vi "Main - 副本.vi"() -> ()   [LabVIEW 2020]
uses:
  System.Windows.Forms
  Global_Variable/Global.vi
  Database/Global1.vi
  <userlib>/_MGI/Menu Building/MenuTypes/MenuStrip/MGI_MenuStrip.lvclass
  <userlib>/_MGI/Menu Building/MenuItemStatusChange/MGI_MenuItemStatusChange.lvclass
panel:
  out "上序状态":string
  in  "表格控件":string[][](table)
  in  "Andon":enum32{"未选择", "缺料报警", "质量报警", "故障报警"}(radio)
  in  "菜单":refnum<k24>(container)
  out "试验计时":u16
  out "工位传感器码":string
  out "生产数量":i32
  out "合格数量":i32
  out "userStatus":string caption="用户状态"
  out "userName":string caption="用户名"
  out "connectionMode":string caption="联机类型"
  out "产品型号":string
  in  "更换产品":refnum<vi>
  out "提示信息":string
  out "错误":bool
  out "时间字符串":string
  out "日期字符串":string
  out "自动":bool
  # "上转向轴组件压装"
  # "实验项目"
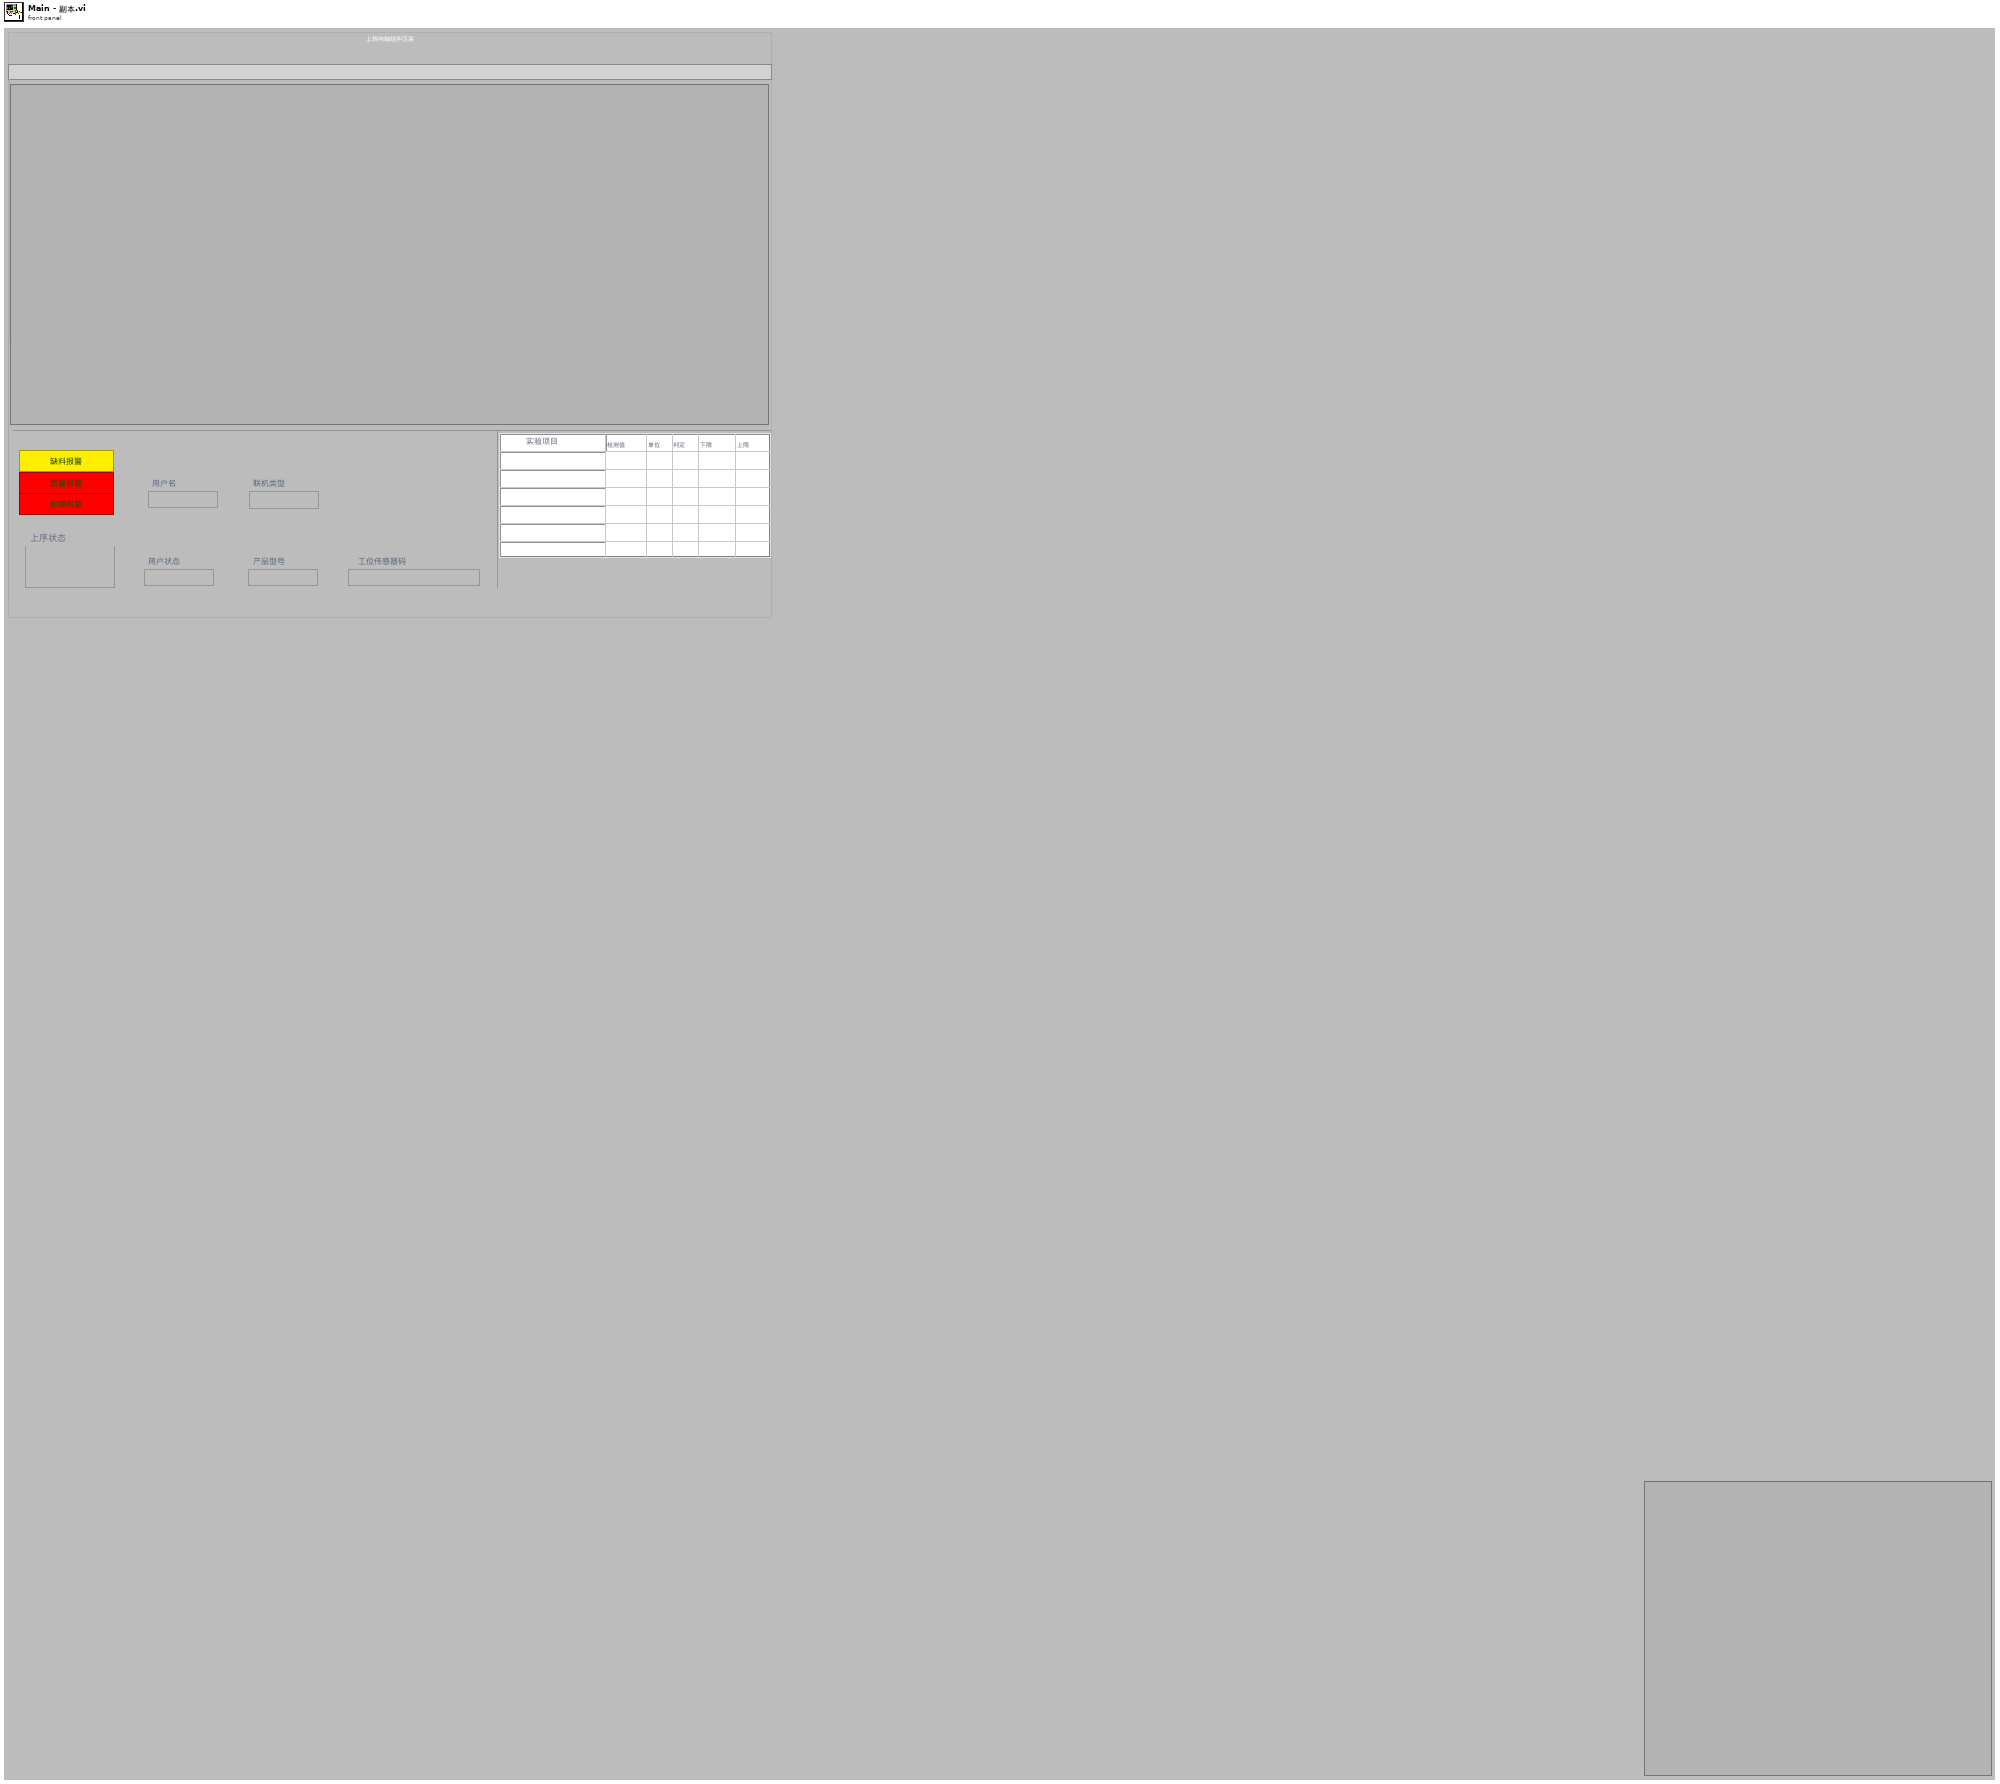
[diagram p1: front panel]
types:
  T1 = enum32{"Invalid", "Standard", "Closed", "Hidden", "Minimized", "Maximized"}
  T2 = cluster{"设备名称":string, "操作人员":string, "设备状态":enum16{"设备离线", "设备正常", "设备缺料", "设备故障", "质量报警"}, "附加信息":string}
  T3 = enum32{"invalid app kind", "Development System", "Run Time System", "Student Edition", "Embedded LabVIEW", "Evaluation", "Custom"}
  T4 = cluster{"用户编号":string, "用户名":string, "用户密码(密文)":string, "用户权限":string}
  T5 = cluster{"Core":cluster{"Current VI Reference":refnum<vi>, "Close Panel on Exit?":bool}, "Your Boolean data":bool, "Your string data":string}
  T6 = cluster{"Current VI Reference":refnum<vi>, "Close Panel on Exit?":bool}
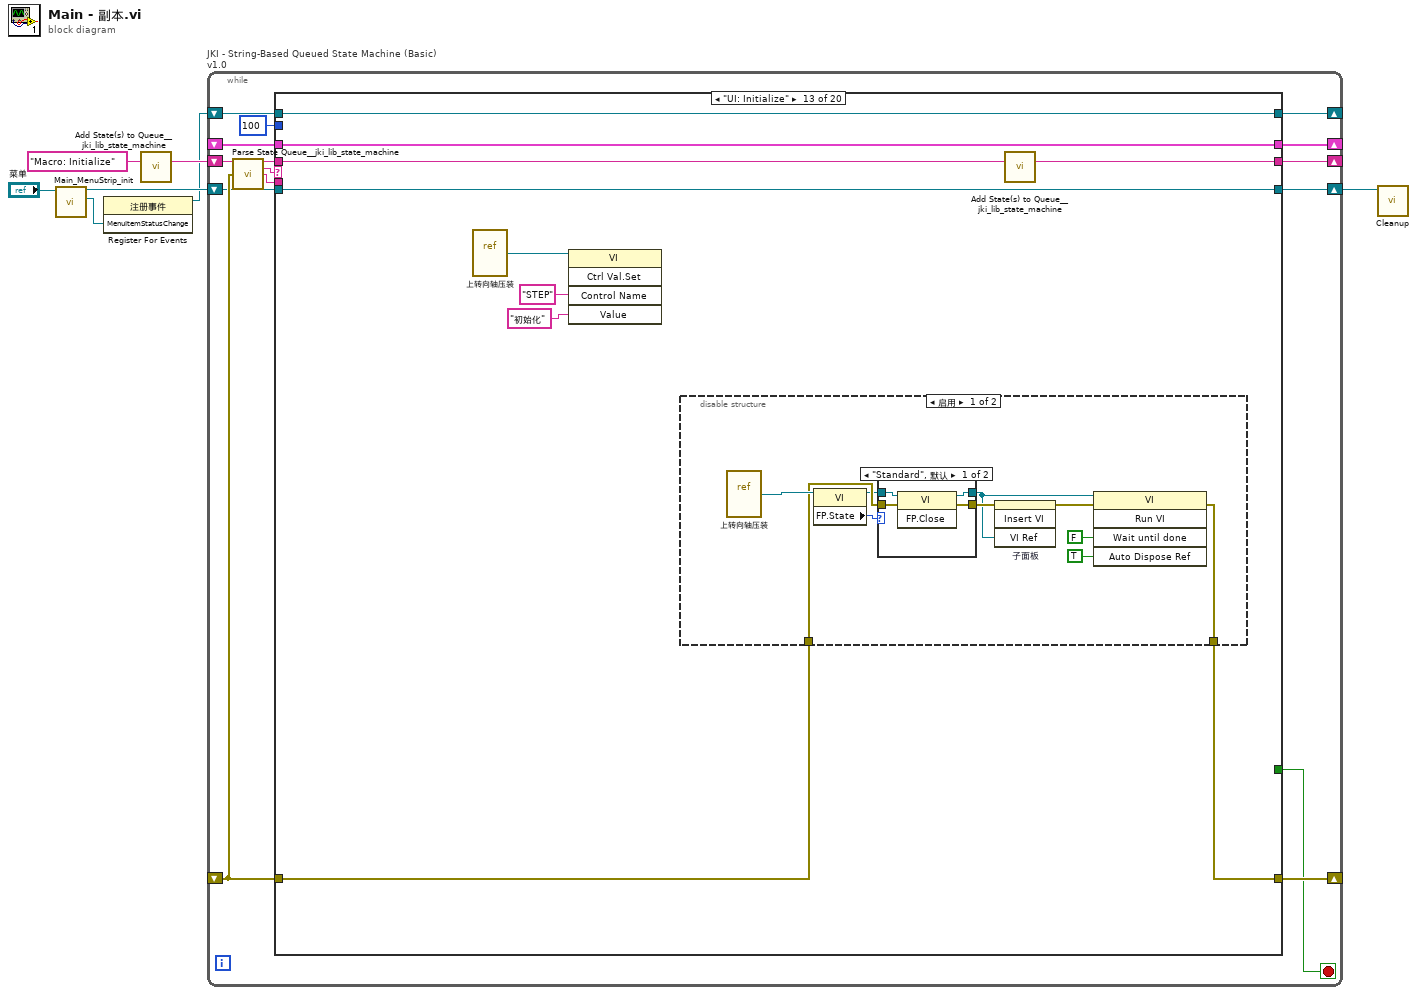
[diagram p0: block diagram]
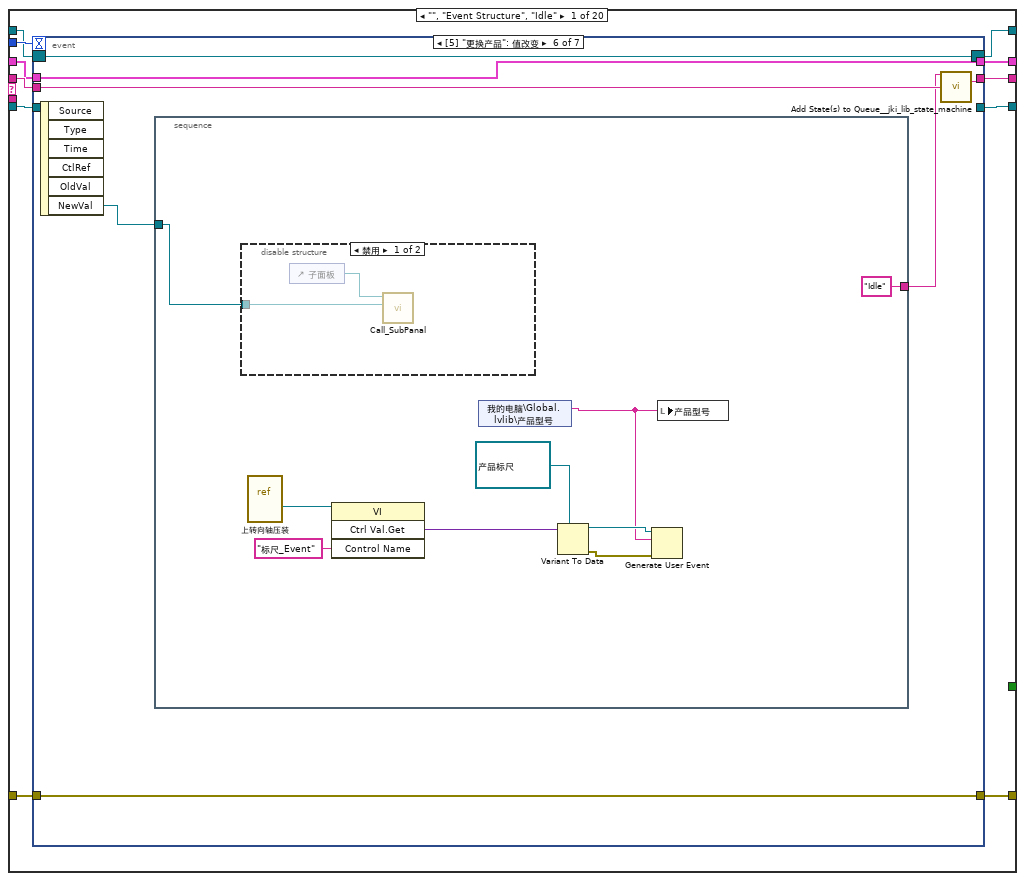
[diagram p2: hidden frame]
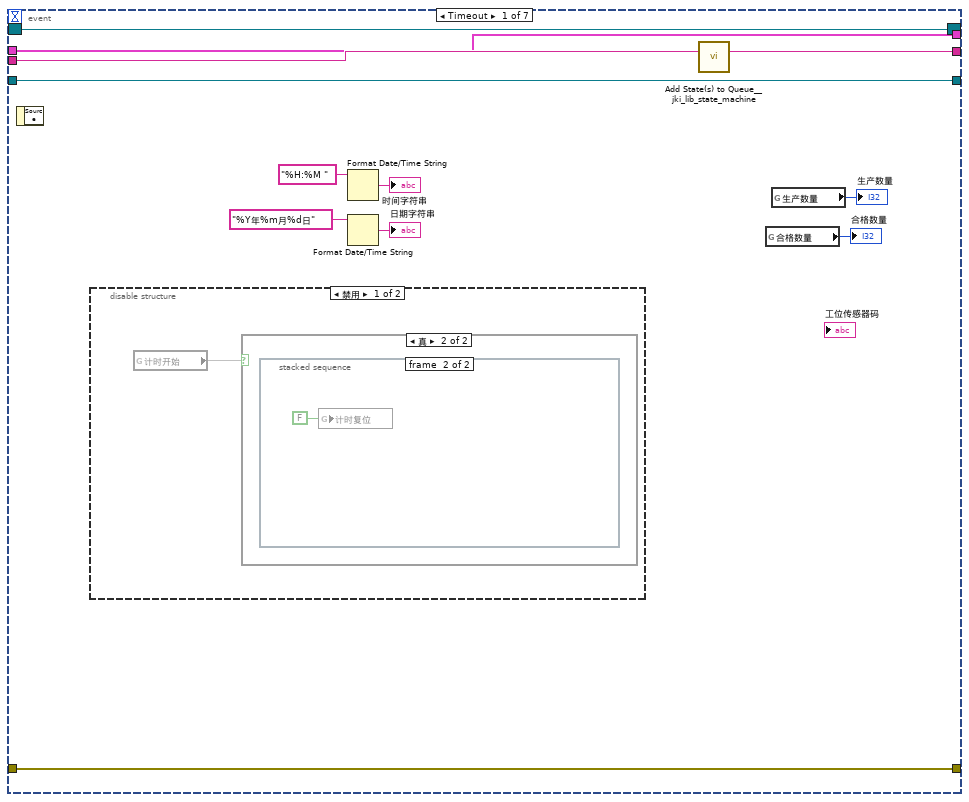
[diagram p3: hidden frame]
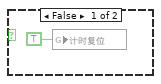
[diagram p4: hidden frame]
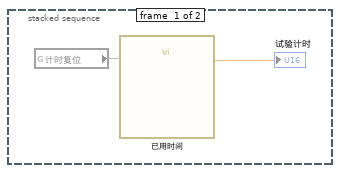
[diagram p5: hidden frame]
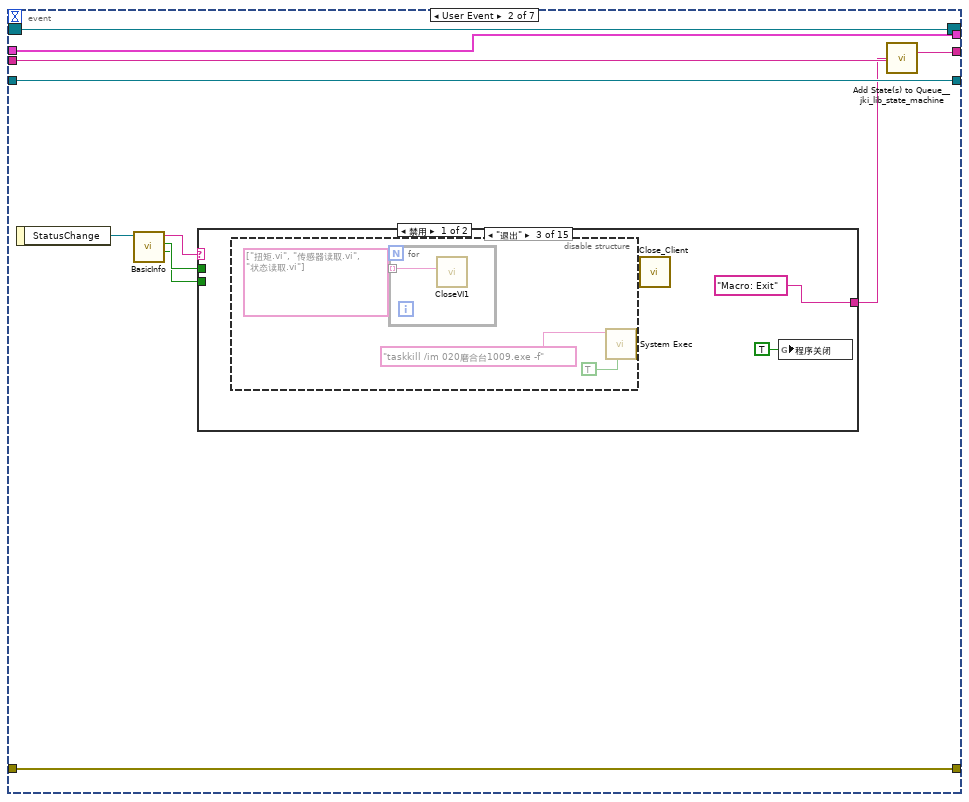
[diagram p7: hidden frame]
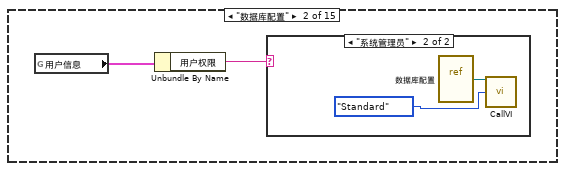
[diagram p9: hidden frame]
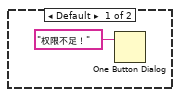
[diagram p10: hidden frame]
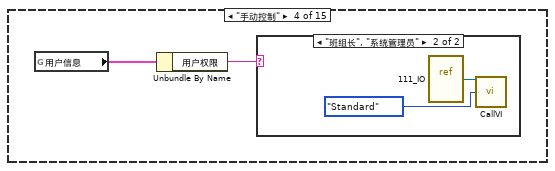
[diagram p12: hidden frame]
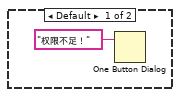
[diagram p13: hidden frame]
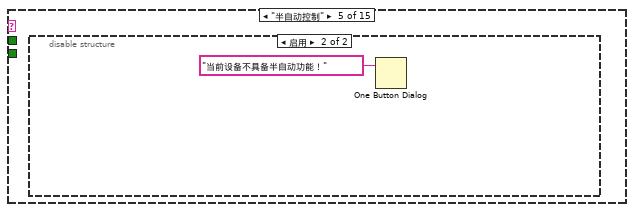
[diagram p14: hidden frame]
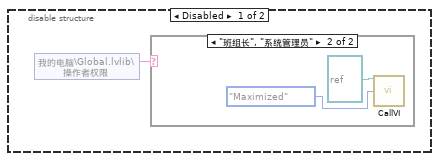
[diagram p15: hidden frame]
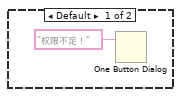
[diagram p16: hidden frame]
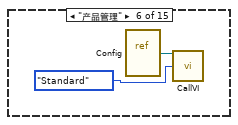
[diagram p17: hidden frame]
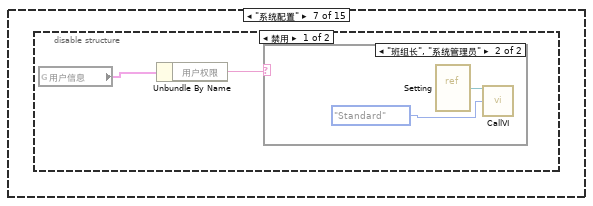
[diagram p18: hidden frame]
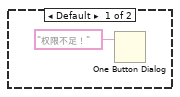
[diagram p19: hidden frame]
diagram:
  n1 = call "Main_MenuStrip_init.vi"("MenuStrip"="菜单") -> ("MenuItemStatusChange"=w2:refnum<user-event>, "Menu out"=w4:refnum<class "MGI_MenuStrip.lvclass">)  [unwired: 9 in]
  n2 = register-events(w2) -> (reference out=w1:refnum<event-registration>)  [unwired: 2 in, 1 out]
  n3 = call <vilib>:"Add State(s) to Queue__jki_lib_state_machine.vi"("State(s) in (\"\")"="Macro: Initialize") -> ("States Out"=w7:string)  [unwired: 14 in]
  n4 = while "JKI - String-Based Queued State Machine (Basic) v1.0" {
    shift-right: [w16] -> _
    shift-left: _ -> [w15]
    shift-right: [w18] -> _
    shift-left: _ -> [w13]
    shift-right: [w17] -> _
    shift-left: w7 -> [w19]
    shift-right: [w11] -> w3
    shift-left: w4 -> [w12]
    shift-right: [w9] -> _
    shift-left: w1 -> [w8]
    stop <- w10 stop-if-true
    n5 = call <vilib>:"Parse State Queue__jki_lib_state_machine.vi"("State Queue"=w19, "Error In (no error)"=w13) -> ("Remaining States"=w21:string, "Current State"=w22:string, "Arguments"=w20:string)  [unwired: 11 in]
    n6 = case shown="\"UI: Initialize\"" w22 {
      selector: w22 -> [_ _ w189 _ _ _ _ _ _ _ _ _ _ _ _ _ _ _ _ _]
      tunnel: w21 -> [w33 w186 w193 w213 w221 w228 w234 w237 w245 w255 w263 w269 w279 w303 w333 w341 w354 w382 w389 w401]
      tunnel: w20 -> [_ _ _ _ _ _ _ _ _ _ _ _ _ _ _ w336 w348 _ _ _]
      tunnel: w15 -> [w31 w183 w191 w204 w218 w226 w231 w238 w242 _ w258 w266 w277 w301 w330 w339 w350 w379 w386 w398]
      tunnel: [w30 w184 w195 w210 errorcluster {"status"=FALSE, "code"=0, "source"=""} ("error out") w225 w232 w235 w243 w252 w259 w267 w276 w299 w331 w337 w351 w380 w387 w399] -> w18
      tunnel: w13 -> [w29 w184 w194 w210 w217 w225 w232 w235 w243 w252 w260 w267 w273 w299 w331 w338 w352 w380 w387 w399]
      tunnel: [w32 w185 w192 w212 w220 w227 w233 w237 w244 w254 w262 w268 w278 w302 w332 w340 w353 w381 w388 w400] -> w17
      tunnel: [w28 w183 w191 w211 w218 w226 w231 w238 w242 w253 w258 w266 w277 w301 w330 w339 w350 w379 w386 w398] -> w16
      tunnel: 100 ("Timeout") -> [w27 _ _ _ _ _ _ _ _ _ _ _ _ _ _ _ _ _ _ _]
      tunnel: w12 -> [w26 w182 w188 w201 w215 w224 w230 w236 w241 w247 w257 w265 w275 w300 w329 w335 w347 w378 w384 w391]
      tunnel: [w25 w182 w188 w201 w215 w224 w230 w236 w241 w247 w257 w265 w275 w300 w329 w335 w347 w378 w384 w391] -> w11
      tunnel: [_ _ _ _ _ TRUE _ _ _ _ _ _ _ _ _ _ _ _ _ _] -> w10
      tunnel: [w23 w181 w187 w200 w214 w222 w229 w239 w240 w248 w256 w264 w274 w298 w326 w334 w346 w377 w383 w390] -> w9
      tunnel: w8 -> [w24 w181 w187 w200 w214 w222 w229 w239 w240 w248 w256 w264 w274 w298 w326 w334 w346 w377 w383 w390]
      frame "", "Event Structure", "Idle" {
        n7 = event shown="[5] \"更换产品\": 值改变" {
          selector: w24 -> [w35 w51 w126 w135 w143 w151 _]
          dyn-events: [w35 w51 w126 w135 w143 w151 _] -> w23
          timeout: w27 -> [_ _ _ _ _ _ _]
          tunnel: w33 -> [w45 w60 w123 w139 w149 w153 w175]
          tunnel: [w44 w58 w124 w140 w148 w154 w175] -> w32
          tunnel: w31 -> [w43 w59 w125 w141 w146 w156 w176]
          tunnel: [w36 w61 w121 w138 w147 w155 w173] -> w30
          tunnel: w29 -> [w36 w61 w121 w138 w147 w155 w173]
          tunnel: [w43 w59 w125 w141 w146 w156 w176] -> w28
          tunnel: w26 -> [w34 w54 w122 _ _ _ w174]
          tunnel: [w34 w54 w122 _ _ _ w174] -> w25
          event Timeout {
            n8 = event-data() -> ()  [unwired: 1 in, 1 out]
            n9 = disable-structure shown="禁用" {
              frame Disabled {
                n10 = global read "Global.vi" "计时开始"() -> (w46)
                n11 = case shown="真" w46 {
                  frame False {
                    n12 = global write "Global.vi" "计时复位"(TRUE ("计时复位")) -> ()
                  }
                  frame True {
                    n13 = stacked-sequence {
                      frame #0 {
                        n14 = global read "Global.vi" "计时复位"() -> (w48)
                        n15 = call "已用时间"("Reset"=w48) -> ("Elapsed Time (s)"=→"试验计时":dbl)  [unwired: 11 in, 7 out]
                      }
                      frame #1 {
                        n16 = global write "Global.vi" "计时复位"(FALSE ("计时复位")) -> ()
                      }
                    }
                  }
                }
              }
              frame Enabled {
              }
            }
            n17 = Format Date/Time String(time format string (%c)="%H:%M ") -> (date/time string=→"时间字符串":string)  [unwired: 2 in]
            n18 = Format Date/Time String(time format string (%c)="%Y年%m月%d日") -> (date/time string=→"日期字符串":string)  [unwired: 2 in]
            n19 = call <vilib>:"Add State(s) to Queue__jki_lib_state_machine.vi"("State(s) in (\"\")"=w45) -> ("States Out"=w44:string)  [unwired: 14 in]
            n20 = global read "Global.vi" "合格数量"() -> (→"合格数量":i32)
            n21 = global read "Global.vi" "生产数量"() -> (→"生产数量":i32)
          }
          event User Event {
            n22 = event-data() -> ("StatusChange"=w52:refnum<class "MGI_MenuItemStatusChange.lvclass">)  [unwired: 1 in]
            n23 = call <userlib>:"BasicInfo.vi"("MGI_MenuItemStatusChange in"=w52) -> ("Enabled?"=w55:bool, "Checked?"=w56:bool, "Tag"=w57:string)  [unwired: 7 in, 1 out]
            n24 = case shown="\"退出\"" w57 {
              tunnel: w56 -> [_ _ _ _ _ _ _ _ _ _ _ _ _ _ _]
              tunnel: w55 -> [_ _ _ _ _ _ _ _ _ _ _ _ _ _ _]
              tunnel: [_ _ "Macro: Exit" _ _ _ _ _ _ _ _ _ _ _ _] -> w53
              frame "假", Default {
              }
              frame "数据库配置" {
                n25 = global read "Global1.vi" "用户信息"() -> (w62:T4)
                n26 = Unbundle By Name(w62) -> ("用户权限"=w63:string)
                n27 = case shown="\"系统管理员\"" w63 {
                  frame Default {
                    n28 = One Button Dialog(message="权限不足！" ("消息")) -> ()  [unwired: 1 in, 1 out]
                  }
                  frame "系统管理员" {
                    n29 = vi-ref "数据库配置.vi"() -> (w66:refnum<vi>)
                    n30 = call "CallVI.vi"("VI引用"=w66, "状态"=T1."Standard") -> ()  [unwired: 11 in, 3 out]
                  }
                }
              }
              frame "退出" {
                n31 = disable-structure shown="禁用" {
                  frame Disabled {
                    n32 = for {
                      tunnel: string[] ["扭矩.vi", "传感器读取.vi", "状态读取.vi"] -> [w72] mode=indexing
                      n33 = call "CloseVI1.vi"("名称或相对路径"=w72) -> ()  [unwired: 10 in, 1 out]
                    }
                    n34 = call <vilib>:"System Exec.vi"("run minimized? (F)"=TRUE, "command line"="taskkill /im 020磨合台1009.exe -f") -> ()  [unwired: 6 in, 4 out]
                  }
                  frame Enabled {
                  }
                }
                n35 = call "Close_Client.vi"() -> ()  [unwired: 12 in]
                n36 = global write "Global.vi" "程序关闭"(TRUE ("程序关闭")) -> ()
              }
              frame "手动控制" {
                n37 = global read "Global1.vi" "用户信息"() -> (w73:T4)
                n38 = Unbundle By Name(w73) -> ("用户权限"=w74:string)
                n39 = case shown="\"班组长\", \"系统管理员\"" w74 {
                  frame Default {
                    n40 = One Button Dialog(message="权限不足！" ("消息")) -> ()  [unwired: 1 in, 1 out]
                  }
                  frame "班组长", "系统管理员" {
                    n41 = vi-ref "111_IO.vi"() -> (w77:refnum<vi>)
                    n42 = call "CallVI.vi"("VI引用"=w77, "状态"=T1."Standard") -> ()  [unwired: 11 in, 3 out]
                  }
                }
              }
              frame "半自动控制" {
                n43 = disable-structure shown="启用" {
                  frame Disabled {
                    n44 = shared-variable "我的电脑\\Global.lvlib\\操作者权限"() -> (w78:string)  [unwired: 1 in, 1 out]
                    n45 = case shown="\"班组长\", \"系统管理员\"" w78 {
                      frame Default {
                        n46 = One Button Dialog(message="权限不足！" ("消息")) -> ()  [unwired: 1 in, 1 out]
                      }
                      frame "班组长", "系统管理员" {
                        n47 = call "CallVI.vi"("VI引用"=refnum<vi> refnum, "状态"=T1."Maximized") -> ()  [unwired: 11 in, 3 out]
                      }
                    }
                  }
                  frame Enabled {
                    n48 = One Button Dialog(message="当前设备不具备半自动功能！" ("消息")) -> ()  [unwired: 1 in, 1 out]
                  }
                }
              }
              frame "产品管理" {
                n49 = vi-ref "Config.vi"() -> (w84:refnum<vi>)
                n50 = call "CallVI.vi"("VI引用"=w84, "状态"=T1."Standard") -> ()  [unwired: 11 in, 3 out]
              }
              frame "系统配置" {
                n51 = disable-structure shown="禁用" {
                  frame Disabled {
                    n52 = global read "Global1.vi" "用户信息"() -> (w85:T4)
                    n53 = Unbundle By Name(w85) -> ("用户权限"=w86:string)
                    n54 = case shown="\"班组长\", \"系统管理员\"" w86 {
                      frame Default {
                        n55 = One Button Dialog(message="权限不足！" ("消息")) -> ()  [unwired: 1 in, 1 out]
                      }
                      frame "班组长", "系统管理员" {
                        n56 = vi-ref "Setting.vi"() -> (w89:refnum<vi>)
                        n57 = call "CallVI.vi"("VI引用"=w89, "状态"=T1."Standard") -> ()  [unwired: 11 in, 3 out]
                      }
                    }
                  }
                  frame Enabled {
                  }
                }
              }
              frame "用户管理" {
                n58 = global read "Global1.vi" "用户信息"() -> (w90:T4)
                n59 = Unbundle By Name(w90) -> ("用户权限"=w91:string)
                n60 = case shown="\"系统管理员\"" w91 {
                  frame Default {
                    n61 = One Button Dialog(message="权限不足！" ("消息")) -> ()  [unwired: 1 in, 1 out]
                  }
                  frame "系统管理员" {
                    n62 = vi-ref "User_manager.vi"() -> (w94:refnum<vi>)
                    n63 = call "CallVI.vi"("VI引用"=w94, "状态"=T1."Standard") -> ()  [unwired: 11 in, 3 out]
                  }
                }
              }
              frame "编码规则" {
                n64 = global read "Global1.vi" "用户信息"() -> (w95:T4)
                n65 = Unbundle By Name(w95) -> ("用户权限"=w96:string)
                n66 = case shown="\"班组长\", \"工艺管理员\", \"系统管理员\"" w96 {
                  frame Default {
                    n67 = One Button Dialog(message="权限不足！" ("消息")) -> ()  [unwired: 1 in, 1 out]
                  }
                  frame "班组长", "工艺管理员", "系统管理员" {
                    n68 = vi-ref "编码规则设置.vi"() -> (w99:refnum<vi>)
                    n69 = call "CallVI.vi"("VI引用"=w99, "状态"=T1."Standard") -> ()  [unwired: 11 in, 3 out]
                  }
                }
              }
              frame "易损件管理" {
                n70 = vi-ref "易损件管理.vi"() -> (w101:refnum<vi>)
                n71 = call "CallVI.vi"("VI引用"=w101, "状态"=T1."Standard") -> ()  [unwired: 11 in, 3 out]
              }
              frame "物料批次管理" {
                n72 = vi-ref "批次管理.vi"() -> (w103:refnum<vi>)
                n73 = call "CallVI.vi"("VI引用"=w103, "状态"=T1."Standard") -> ()  [unwired: 11 in, 3 out]
              }
              frame "报表" {
                n74 = call "文件对话框"("start path"=path "D:/report", "prompt"="打开报表", "pattern (all files)"="*.doc;*.docx", "pattern label"="Word 文档") -> ("selected path"=w104:path, "error out"=w105:errorcluster)  [unwired: 8 in, 2 out]
                n75 = case shown="无错误" w105 {
                  selector: w105 -> [w111 w113]
                  tunnel: w104 -> [w112 _]
                  frame No Error {
                    w110 = 1 items=["Normal", "Maximize", "Minimize"] ("cpubbs_WindowState")
                    n76 = call "Open_Word.vi"("File Path"=w112, "cpubbs_WindowState"=w110, "错误输入（无错误）"=w111) -> ()  [unwired: 12 in, 1 out]
                  }
                  frame Error {
                    n77 = call <vilib>:"Clear Errors.vi"("error in (no error)"=w113) -> ()  [unwired: 5 in, 2 out]
                  }
                }
              }
              frame "报警信息" {
                n78 = vi-ref "报警信息.vi"() -> (w115:refnum<vi>)
                n79 = call "CallVI.vi"("VI引用"=w115, "状态"=T1."Standard") -> ()  [unwired: 11 in, 3 out]
              }
              frame "关于" {
                n80 = vi-ref "About.vi"() -> (w117:refnum<vi>)
                n81 = call "CallVI.vi"("VI引用"=w117, "状态"=T1."Standard") -> ()  [unwired: 11 in, 3 out]
              }
              frame "操作演示" {
                n82 = call <vilib>:"Application Directory.vi"() -> ("Application Directory"=w120:path)
                n83 = Build Path(base path=w120, name or relative path="操作演示" ("名称或相对路径")) -> (appended path=w119:path)
                n84 = call "自动播放ppt.vi"("路径"=w119) -> ()  [unwired: 10 in, 1 out]
              }
            }
            n85 = call <vilib>:"Add State(s) to Queue__jki_lib_state_machine.vi"("State(s) in (\"\")"=w60, "State(s) at Back (\"\")"=w53) -> ("States Out"=w58:string)  [unwired: 13 in]
          }
          event "自动": Mouse Down {
            n86 = event-data() -> ()  [unwired: 1 in, 1 out]
            n87 = disable-structure shown="禁用" {
              frame Disabled {
                n88 = local read "自动"() -> (w127:bool)
                n89 = case shown="假" w127 {
                  frame False {
                    n90 = call "设备状态.vi"() -> ("Status_Read"=w128:i16)  [unwired: 11 in]
                    n91 = case shown="5" w128 {
                      frame 0, Default {
                        n92 = One Button Dialog(message="请复位！" ("消息")) -> ()  [unwired: 1 in, 1 out]
                      }
                      frame 5 {
                      }
                    }
                  }
                  frame True {
                    n93 = Two Button Dialog(message="确定要退出自动？" ("消息")) -> (T button?=w130:bool)  [unwired: 2 in]
                    n94 = case shown="真" w130 {
                      frame False {
                      }
                      frame True {
                        n95 = vi-ref "Auto.vi"() -> (w134:refnum<vi>)
                        n96 = invoke class="VI" method="Ctrl Val.Set"(reference=w134, "Control Name"="STEP" ("控件名"), "Value"="退出自动" ("控件名")) -> ()  [unwired: 2 in, 5 out]
                      }
                    }
                  }
                }
              }
              frame Enabled {
              }
            }
            n97 = call <vilib>:"Add State(s) to Queue__jki_lib_state_machine.vi"("State(s) in (\"\")"=w123) -> ("States Out"=w124:string)  [unwired: 14 in]
          }
          event "错误": Mouse Down {
            n98 = event-data() -> ()  [unwired: 1 in, 8 out]
            n99 = vi-ref "报警信息.vi"() -> (w137:refnum<vi>)
            n100 = call "CallVI.vi"("VI引用"=w137, "状态"=T1."Standard") -> ()  [unwired: 11 in, 3 out]
            n101 = call <vilib>:"Add State(s) to Queue__jki_lib_state_machine.vi"("State(s) in (\"\")"=w139) -> ("States Out"=w140:string)  [unwired: 14 in]
          }
          event Panel Close? {
            w142 = TRUE ("程序关闭")
            n102 = event-data() -> ()  [unwired: 1 in, 1 out]
            n103 = global write "Global.vi" "程序关闭"(w142) -> ()
            n104 = call <vilib>:"Add State(s) to Queue__jki_lib_state_machine.vi"("State(s) in Front (\"\")"="S7: Stop\nMacro: Exit", "State(s) in (\"\")"=w149) -> ("States Out"=w148:string)  [unwired: 13 in]
            n105 = Quit LabVIEW(quit? (T)=w142) -> ()
            n106 = event-data("Discard?"=TRUE) -> ()  [unwired: 1 in, 1 out]
          }
          event "更换产品": Value Change {
            n107 = event-data() -> ("NewVal"=w152:refnum<vi>)  [unwired: 1 in, 5 out]
            n108 = stacked-sequence {
              tunnel: w152 -> [w165]
              tunnel: ["Idle"] -> w150
              frame #0 {
                n109 = disable-structure shown="禁用" {
                  disable-tunnel: w165 -> [w167 _]
                  frame Disabled {
                    n110 = control-ref of="子面板"() -> (w166:refnum<vi>)
                    n111 = call "Call_SubPanal.vi"("VI引用句柄"=w167, "SubPnl引用句柄"=w166) -> ()  [unwired: 9 in, 1 out]
                  }
                  frame Enabled {
                  }
                }
                n112 = vi-ref "上转向轴压装.vi"() -> (w162:refnum<vi>)
                n113 = invoke class="VI" method="Ctrl Val.Get"(reference=w162, "Control Name"="标尺_Event" ("控件名")) -> ("Get Control Value Variant"=w161:variant)  [unwired: 2 in, 3 out]
                n114 = shared-variable "我的电脑\\Global.lvlib\\产品型号"() -> (w157:string)  [unwired: 1 in, 1 out]
                n115 = Variant To Data(type=refnum<user-event> refnum ("标尺_Event"), Variant=w161) -> (data=w158:refnum<user-event>, error out=w159:errorcluster)  [unwired: 1 in]
                n116 = Generate User Event(user event=w158, event data cluster=w157, error in=w159) -> ()  [unwired: 1 in, 2 out]
                n117 = local write "产品型号"(w157) -> ()
              }
            }
            n118 = call <vilib>:"Add State(s) to Queue__jki_lib_state_machine.vi"("State(s) in Front (\"\")"=w150, "State(s) in (\"\")"=w153) -> ("States Out"=w154:string)  [unwired: 13 in]
          }
          event "Andon": Value Change {
            n119 = event-data() -> ("NewVal"=w172:enum32{"未选择", "缺料报警", "质量报警", "故障报警"})  [unwired: 1 in]
            n120 = case shown="\"故障报警\"" w172 {
              tunnel: [enum16{"设备离线", "设备正常", "设备缺料", "设备故障", "质量报警"}."设备正常" ("设备状态") enum16{"设备离线", "设备正常", "设备缺料", "设备故障", "质量报警"}."设备缺料" ("设备状态") enum16{"设备离线", "设备正常", "设备缺料", "设备故障", "质量报警"}."质量报警" ("设备状态") enum16{"设备离线", "设备正常", "设备缺料", "设备故障", "质量报警"}."设备故障" ("设备状态")] -> w170
              frame "未选择", Default {
              }
              frame "缺料报警" {
              }
              frame "质量报警" {
              }
              frame "故障报警" {
              }
            }
            n121 = local read "userName"() -> (w169:string)
            n122 = Bundle By Name(cluster=T2 {"设备名称"="上转向轴组件装配", "操作人员"="", "设备状态"=enum."设备离线", "附加信息"=""} ("设备信息"), "操作人员"=w169, "设备状态"=w170) -> (w168:T2)
            n123 = call "Change_Client.vi"("设备信息"=w168) -> ()  [unwired: 10 in, 1 out]
          }
        }
      }
      frame "---------- Core ----------" {
        n124 = call <vilib>:"Add State(s) to Queue__jki_lib_state_machine.vi"("State(s) in (\"\")"=w186) -> ("States Out"=w185:string)  [unwired: 14 in]
      }
      frame Default {
        w198 = 42 items=["No error", "Argument error", "Memory is full", "Out of zone", "End of file", "File already open", "Generic file I/O error", "File not found", "File permission error", "Disk is full", "Duplicate path", "Too many files open", "System feature not enabled", "Resource file not found", "Cannot add resource", "Resource not found", "Image not found", "Image memory error", "Pen does not exist", "Config type invalid", "Config token not found", "Config parse error", "Config memory error", "Bad external code format", "Bad external code offset", "External code not present", "Null window", "Destroy window error", "Null menu", "Print aborted", "Bad print record", "Print driver error", "Windows error during printing", "Memory error during printing", "Print dialog error", "Generic print error", "Invalid device refnum", "Device not found", "Device parameter error", "Device unit error", "Cannot open device", "Device call aborted", "Generic error", "Cancelled by user", "Object ID too low", "Object ID too high", "Object not in heap", "Unknown heap", "Unknown object (invalid DefProc)", "Unknown object (DefProc not in table)", "Message out of range", "Invalid (null) method", "Unknown message", "Manager call not supported", "Bad address", "Network operation in progress", "Network operation timed out", "Connection is busy", "Network attribute not supported", "Network error", "Address in use", "System out of memory", "Connection aborted", "Connection refused", "Not connected", "Already connected", "Connection closed", "Initialization error (interapplication manager)", "Bad occurrence", "Wait on unbound occurrence handler", "Occurrence queue overflow", "Datalog type conflict", "Unused", "Unrecognized type (interapplication manager)", "Memory corrupt", "Failed to make temporary DLL", "Old CIN version", "Drag socket not found", "Failed to load drop-object", "Failed to register OLE object", "Failed to release OLE object", "Format specifier type mismatch", "Unknown format specifier", "Too few format specifiers", "Too many format specifiers", "Scan failed", "Newer CIN version", "Error converting to variant", "Runtime menu error", "Password tampered", "Variant attribute not found", "Incompatible variant data type", "Event data is not available", "Event Store is not present", "Occurrence is not found", "Event Queue is not created", "Event info is not available", "Refnum passed is NULL", "Error retrieving Class GUID", "Error retrieving CoClass GUID", "Error retrieving TypeLib GUID.", "Bad built application magic bytes.", "Specific driver is different from the specific driver associated with the Logical Name.", "There is no session opened to the class driver.", "Max Error", "MAX - Error with config objects", "MAX - Error loading configuration", "MAX - Group not supported"]
        # "Current State"
        n125 = Format Into String(format string="Software Exception: Unhandled State \"%s\"." ("message"), error in=w194, w189) -> (resulting string=w197:string, error out=w196:errorcluster)  [unwired: 1 in]
        n126 = call <vilib>:"Error Cluster From Error Code.vi"("show call chain? (False)"=TRUE, "error in (no error)"=w196, "error message (\"\")"=w197, "error code (0)"=w198) -> ("error out"=w195:errorcluster)  [unwired: 5 in]
        n127 = call <vilib>:"Add State(s) to Queue__jki_lib_state_machine.vi"("State(s) in (\"\")"=w193) -> ("States Out"=w192:string)  [unwired: 14 in]
      }
      frame "Initialize Core Data" {
        # "originally closed?"
        # "exe?"
        n128 = property class="VI"() -> ("Front Panel.Open"=w209:bool)  [unwired: 2 in, 2 out]
        n129 = property class="App"() -> ("App.Kind"=w208:T3)  [unwired: 2 in, 2 out]
        n130 = control-ref of="Current VI Reference"() -> (w202:refnum<vi>)
        n131 = Not(x=w209) -> (.not. x?=w206:bool)
        n132 = Equal?(x=w208, y=T3."Run Time System" ("Application:Kind")) -> (x = y?=w205:bool)
        n133 = Or(x=w206, y=w205) -> (x .or. y?=w203:bool)
        n134 = Bundle By Name(cluster=w204, "Core.Current VI Reference"=w202, "Core.Close Panel on Exit?"=w203) -> (w211:T5)
        n135 = call <vilib>:"Add State(s) to Queue__jki_lib_state_machine.vi"("State(s) in (\"\")"=w213) -> ("States Out"=w212:string)  [unwired: 14 in]
      }
      frame "Error Handler" {
        n136 = call <vilib>:"General Error Handler.vi"("error in (no error)"=w217) -> ()  [unwired: 10 in, 5 out]
        n137 = call <vilib>:"Add State(s) to Queue__jki_lib_state_machine.vi"("State(s) in Front (\"\")"="/* Post Error States", "State(s) in (\"\")"=w221) -> ("States Out"=w220:string)  [unwired: 13 in]
      }
      frame "Exit" {
        n138 = call <vilib>:"Add State(s) to Queue__jki_lib_state_machine.vi"("State(s) in (\"\")"=w228) -> ("States Out"=w227:string)  [unwired: 14 in]
        n139 = Quit LabVIEW() -> ()  [unwired: 1 in]
      }
      frame "--------- Library --------" {
        n140 = call <vilib>:"Add State(s) to Queue__jki_lib_state_machine.vi"("State(s) in (\"\")"=w234) -> ("States Out"=w233:string)  [unwired: 14 in]
      }
      frame "S7: Initialize" {
      }
      frame "---------- Data ----------" {
        n141 = call <vilib>:"Add State(s) to Queue__jki_lib_state_machine.vi"("State(s) in (\"\")"=w245) -> ("States Out"=w244:string)  [unwired: 14 in]
      }
      frame "Data: Initialize" {
        (unwired) FALSE ("计时结束")
        w249 = T6 {"Current VI Reference"=refnum, "Close Panel on Exit?"=FALSE}  # Core
        w251 = TRUE  # Your Boolean data
        w250 = ""  # Your string data
        n142 = global write "Global.vi" "程序关闭"(FALSE ("程序关闭")) -> ()
        n143 = Bundle("Core"=w249, "Your Boolean data"=w251, "Your string data"=w250) -> (w253:T5)  [unwired: 1 in]
        n144 = call <vilib>:"Add State(s) to Queue__jki_lib_state_machine.vi"("State(s) in (\"\")"=w255) -> ("States Out"=w254:string)  [unwired: 14 in]
      }
      frame "Data: Cleanup" {
        n145 = Unbundle By Name(w258) -> ("Core.Current VI Reference"=w261:refnum<vi>)
        n146 = Close Reference(reference=w261, error in (no error)=w260) -> (error out=w259:errorcluster)
        n147 = call <vilib>:"Add State(s) to Queue__jki_lib_state_machine.vi"("State(s) in (\"\")"=w263) -> ("States Out"=w262:string)  [unwired: 14 in]
      }
      frame "---------- UI ----------" {
        # "Do not put any code in this frame.\n(It is a separator no-op. You can make a copy of this frame to create a new UI frame)"
        n148 = call <vilib>:"Add State(s) to Queue__jki_lib_state_machine.vi"("State(s) in (\"\")"=w269) -> ("States Out"=w268:string)  [unwired: 14 in]
      }
      frame "UI: Initialize" {
        n149 = vi-ref "上转向轴压装.vi"() -> (w272:refnum<vi>)
        n150 = invoke class="VI" method="Ctrl Val.Set"(reference=w272, "Control Name"="STEP" ("控件名"), "Value"="初始化" ("控件名")) -> ()  [unwired: 2 in, 5 out]
        n151 = disable-structure shown="启用" {
          disable-tunnel: [w286 _] -> w276
          disable-tunnel: w273 -> [w284 _]
          frame Enabled {
            n152 = vi-ref "上转向轴压装.vi"() -> (w285:refnum<vi>)
            n153 = property class="VI"(reference=w285) -> (reference out=w283:refnum<vi>, "FP.State"=w282:T1)  [unwired: 1 in, 1 out]
            n154 = case shown="\"Standard\", 默认" w282 {
              tunnel: w284 -> [w292 w294]
              tunnel: w283 -> [w293 w295]
              tunnel: [w291 w295] -> w280
              tunnel: [w290 w294] -> w281
              frame "Standard", Default {
                n155 = invoke class="VI" method="FP.Close"(reference=w293, error in=w292) -> (reference out=w291:refnum<vi>, error out=w290:errorcluster)  [unwired: 1 in, 1 out]
              }
              frame "Invalid", "Closed" {
              }
            }
            n156 = invoke on="子面板" class="SubPnl" method="Insert VI"(error in=w281, "VI Ref"=w280) -> (error out=w289:errorcluster)  [unwired: 2 in, 3 out]
            n157 = invoke class="VI" method="Run VI"(reference=w280, error in=w289, "Wait until done"=FALSE ("结束前等待"), "Auto Dispose Ref"=TRUE ("自动销毁引用")) -> (error out=w286:errorcluster)  [unwired: 1 in, 4 out]
          }
          frame Disabled {
            n158 = vi-ref "Auto.vi"() -> (w297:refnum<vi>)
            n159 = call "CallVI.vi"("VI引用"=w297, "状态"=T1."Maximized") -> ()  [unwired: 11 in, 3 out]
          }
        }
        n160 = call <vilib>:"Add State(s) to Queue__jki_lib_state_machine.vi"("State(s) in (\"\")"=w279) -> ("States Out"=w278:string)  [unwired: 14 in]
      }
      frame "UI: Init" {
        n161 = stacked-sequence {
          tunnel: w299 -> [_ _ _ _]
          frame #0 {
            n162 = global write "Global.vi" "程序关闭"(FALSE ("程序关闭")) -> ()
          }
          frame #1 {
            w311 = 0
            n163 = shared-variable "我的电脑\\Global.lvlib\\总成追溯码"("   " ("工位追溯码")) -> ()  [unwired: 1 in, 1 out]
            n164 = global write "Global.vi" "生产数量"(w311) -> ()
            n165 = global write "Global.vi" "合格数量"(w311) -> ()
            n166 = global read "Global1.vi" "用户信息"() -> (w306:T4)
            n167 = global read "Global1.vi" "联机模式"() -> (w305:enum16{"单机", "追溯"})
            n168 = Unbundle By Name(w306) -> ("用户名"=→"userName":string, "用户权限"=→"userStatus":string)
            n169 = case shown="\"追溯\"" w305 {
              tunnel: ["联网" ("connectionMode") "单机" ("connectionMode")] -> w312
              frame "追溯" {
              }
              frame "单机", Default {
              }
            }
            "connectionMode" <- w312
            "产品型号" <- "" ("产品型号")
          }
          frame #2 {
            n170 = control-ref of="表格控件"() -> (w315:refnum<vi>)
            n171 = control-ref of="提示信息"() -> (w317:refnum<vi>)
            n172 = control-ref of="自动"() -> (w318:refnum<vi>)
            n173 = control-ref of="错误"() -> (w319:refnum<vi>)
            n174 = control-ref of="更换产品"() -> (w316:refnum<vi>)
            n175 = global write "Global.vi" "提示信息"(w317) -> ()
            n176 = global write "Global.vi" "程序自动"(w318) -> ()
            n177 = global write "Global.vi" "报警图标"(w319) -> ()
            n178 = global write "Global.vi" "Result"(w315) -> ()
            n179 = global write "Global.vi" "更换产品"(w316) -> ()
          }
          frame #3 {
            w320 = -2
            n180 = global read "Global.vi" "Result"() -> (w323:refnum<vi>)
            n181 = property class="Tbl"(reference=w323, "Row Headers[]"=string[] [], "Value"=string[][] []) -> ()  [unwired: 1 in, 2 out]
            n182 = Bundle(w320, w320) -> (w321:cluster{i32, i32})  [unwired: 1 in]
            n183 = call "Start_Client.vi"() -> ()  [unwired: 12 in]
            n184 = property class="Tbl"(reference=w323, "Active Cell"=w321, "Cell BG Color"=u32 16777216 ("活动单元格:单元格背景色")) -> ()  [unwired: 1 in, 2 out]
          }
        }
        n185 = call <vilib>:"Add State(s) to Queue__jki_lib_state_machine.vi"("State(s) in (\"\")"=w303) -> ("States Out"=w302:string)  [unwired: 14 in]
      }
      frame "UI: Config" {
        n186 = vi-ref "Config.vi"() -> (w328:refnum<vi>)
        n187 = call "CallVI.vi"("VI引用"=w328, "状态"=T1."Standard") -> ()  [unwired: 11 in, 3 out]
        n188 = call <vilib>:"Add State(s) to Queue__jki_lib_state_machine.vi"("State(s) in (\"\")"=w333) -> ("States Out"=w332:string)  [unwired: 14 in]
      }
      frame "UI: Cursor Set" {
        # "Argument"
        n189 = case shown="\"Idle\", 默认" w336 {
          tunnel: w338 -> [w343 w345]
          tunnel: [w342 w344] -> w337
          frame "Idle", Default {
            n190 = call <vilib>:"Unset Busy.vi"("error in (no error)"=w343) -> ("error out"=w342:errorcluster)  [unwired: 10 in]
          }
          frame "Busy" {
            n191 = call <vilib>:"Set Busy.vi"("error in (no error)"=w345) -> ("error out"=w344:errorcluster)  [unwired: 9 in, 1 out]
          }
        }
        n192 = call <vilib>:"Add State(s) to Queue__jki_lib_state_machine.vi"("State(s) in (\"\")"=w341) -> ("States Out"=w340:string)  [unwired: 14 in]
      }
      frame "UI: Front Panel State" {
        # "Argument"
        n193 = Unbundle By Name(w350) -> ("Core.Current VI Reference"=w349:refnum<vi>)
        n194 = case shown="\"Close\"" w348 {
          tunnel: w352 -> [w358 w371]
          tunnel: [w360 w372] -> w351
          tunnel: w349 -> [w359 w369]
          frame "Open", Default {
            n195 = property class="VI"(reference=w359, error in=w358) -> (reference out=w356:refnum<vi>, error out=w357:errorcluster, "Front Panel.Open"=w355:bool)
            n196 = case shown="假" w355 {
              tunnel: [w363 w366] -> w360
              tunnel: w357 -> [w362 w366]
              tunnel: w356 -> [w361 _]
              frame False {
                n197 = invoke class="VI" method="FP.Open"(reference=w361, error in=w362, "Activate"=TRUE, "State"=T1."Standard") -> (error out=w363:errorcluster)  [unwired: 1 in, 4 out]
              }
              frame True {
              }
            }
          }
          frame "Close" {
            n198 = property class="VI"(reference=w369, error in=w371) -> (reference out=w368:refnum<vi>, error out=w370:errorcluster, "Front Panel.Open"=w367:bool)
            n199 = case shown="真" w367 {
              tunnel: [w373 w376] -> w372
              tunnel: w370 -> [w373 w375]
              tunnel: w368 -> [_ w374]
              frame False {
              }
              frame True {
                n200 = invoke class="VI" method="FP.Close"(reference=w374, error in=w375) -> (error out=w376:errorcluster)  [unwired: 1 in, 2 out]
              }
            }
          }
        }
        n201 = call <vilib>:"Add State(s) to Queue__jki_lib_state_machine.vi"("State(s) in (\"\")"=w354) -> ("States Out"=w353:string)  [unwired: 14 in]
      }
      frame "---------- Macro ----------" {
        n202 = call <vilib>:"Add State(s) to Queue__jki_lib_state_machine.vi"("State(s) in (\"\")"=w382) -> ("States Out"=w381:string)  [unwired: 14 in]
      }
      frame "Macro: Initialize" {
        n203 = call <vilib>:"Add State(s) to Queue__jki_lib_state_machine.vi"("State(s) in Front (\"\")"="Data: Initialize\nInitialize Core Data\nS7: Initialize\nIdle\nUI: Init\nUI: Front Panel State >> Open\nUI: Initialize\nUI: Config", "State(s) in (\"\")"=w389) -> ("States Out"=w388:string)  [unwired: 13 in]
      }
      frame "Macro: Exit" {
        n204 = Unbundle By Name(w398) -> ("Core.Close Panel on Exit?"=w397:bool)
        n205 = Select(t="UI: Front Panel State >> Close", s=w397, f="") -> (s? t:f=w394:string)
        n206 = call <vilib>:"Add State(s) to Queue__jki_lib_state_machine.vi"("State(s) in (\"\")"=w394, "State(s) at Back (\"\")"="Data: Cleanup\nExit") -> ("States Out"=w392:string)  [unwired: 13 in]
        n207 = call <vilib>:"Add State(s) to Queue__jki_lib_state_machine.vi"("State(s) in Front (\"\")"=w392, "State(s) in (\"\")"=w401) -> ("States Out"=w400:string)  [unwired: 13 in]
      }
    }
  }
  n208 = call-dynamic "Cleanup.vi"("MenuStrip in"=w3) -> ()  [unwired: 10 in, 1 out]
